vi "UHR-Fleezers Control (host) - 12.8.1.vi"() -> ()   [LabVIEW 2012] (continued)
              }
            }
          }
        }
      }
      event "Stop All": Value Change {
        # "Stopping blue laser before shutting off program"
        n823 = event-data() -> ()  [unwired: 1 in, 5 out]
        n824 = local read "Delay (ms)"() -> (w1275:i32)
        n825 = call "serial write macro.vi"("String"="l0", "Delay (ms)"=w1275, "VISA resource name"=w1278) -> ("read buffer"=w1273:string, "error out"=w1274:errorcluster, "VISA resource name out"=w1277:refnum<visa-resource-name>)
        n826 = local write "read blue buffer"(w1273) -> ()
        n827 = local write "Blue Error Out"(w1274) -> ()
        n828 = VISA Close(VISA resource name=w1277) -> ()  [unwired: 1 in, 1 out]
        n829 = local read "Stop All"() -> (w1279:bool)
      }
    }
    n830 = node-c288() -> ()  [unwired: 1 in, 1 out]
  }
  n831 = node-c288(2 ("Processor")) -> (w78:T27)  [unwired: 3 out]
  n832 = node-c288() -> (w34:T27)  [unwired: 4 out]
  n833 = node-c288() -> (w80:T27)  [unwired: 4 out]
  n834 = while "Duncan's play event loop" {
    stop <- w1281 stop-if-true
    n835 = Create User Event(user event datatype=TRUE ("Boolean")) -> (user event=w1282:refnum<user-event>)  [unwired: 1 in, 1 out]
    n836 = Create User Event(user event datatype=TRUE ("Boolean")) -> (user event=w1289:refnum<user-event>)  [unwired: 1 in, 1 out]
    n837 = global write "Global for fluorescence simulation mean (30 samples), (power series).vi" "Red Signal"(w1282) -> ()
    n838 = global write "Global for fluorescence simulation mean (30 samples), (power series).vi" "Green Signal"(w1289) -> ()
    n839 = register-events(w1289, w1282) -> (reference out=w1288:refnum<event-registration>)  [unwired: 2 in, 1 out]
    n840 = event shown="[1] \"Get Fluorophore\": Value Change" {
      selector: w1288 -> [_ _ _ _]
      dyn-events: _ -> [_ _ _ _]
      timeout: 100 -> [_ _ _ _]
      event Timeout {
        n841 = event-data() -> ()  [unwired: 1 in, 2 out]
      }
      event "Get Fluorophore": Value Change {
        n842 = event-data() -> ("OldVal"=w1291:bool)  [unwired: 1 in, 4 out]
        n843 = case shown="True" w1291 {
          selector: w1291 -> [_ w1292]
          frame False {
          }
          frame True {
            n844 = property on="Move to Position 3" class="Bool"("Val(Sgnl)"=w1292) -> ()  [unwired: 2 in, 2 out]
            n845 = case shown="1" "Numeric" {
              frame 0, Default {
              }
              frame 1 {
                n846 = property on="Green Laser ON" class="Bool (strict)"("Val(Sgnl)"=TRUE ("Value (Signaling)")) -> ()  [unwired: 2 in, 2 out]
              }
              frame 2 {
                n847 = property on="Red Laser ON" class="Bool (strict)"("Val(Sgnl)"=TRUE) -> ()  [unwired: 2 in, 2 out]
              }
            }
          }
        }
      }
      event User Event {
        n848 = event-data() -> ("Boolean"=w1296:bool)  [unwired: 1 in, 3 out]
        "Green Fluorophore" <- w1296
        n849 = property on="Get Fluorophore" class="Bool (strict)"("Val(Sgnl)"=w1296) -> ()  [unwired: 2 in, 2 out]
      }
      event User Event {
        n850 = event-data() -> ("Boolean"=w1297:bool)  [unwired: 1 in, 3 out]
        "Red Fluorophore" <- w1297
        n851 = property on="Get Fluorophore" class="Bool (strict)"("Val(Sgnl)"=w1297) -> ()  [unwired: 2 in, 2 out]
      }
    }
    n852 = property on="Get Fluorophore" class="Bool (strict)"("Val(Sgnl)"="Get Fluorophore") -> ()  [unwired: 2 in, 2 out]
    n853 = Wait (ms)(milliseconds to wait=u32 100) -> ()  [unwired: 1 out]
    n854 = local read "Stop All"() -> (w1280:bool)
    n855 = Or(x=w1280, y="stop") -> (x .or. y?=w1281:bool)
  }
  n856 = timed-loop "Basic control parameters (all FPGA settings, other basic controls)" {
    shift-right: [w1305] -> _
    shift-left: errorcluster {"status"=FALSE, "code"=0, "source"=""} ("error out") -> [_]
    tunnel: [w1304] -> _
    timing: w78 -> [_]
    timing-out: [_] -> w77
    tunnel: w54 -> [w1303]
    tunnel: w44 -> [w1302]
    tunnel: w43 -> [w1301]
    tunnel: w42 -> [w1300]
    tunnel: w41 -> [w1299]
    tunnel: w17 -> [w1298]
    stop <- w1304 stop-if-true
    n857 = node-c288() -> ()  [unwired: 2 out]
    n858 = event shown="[32] \"Read Cal\": Value Change" {
      selector: _ -> [_ _ _ _ _ _ _ _ _ _ _ _ _ _ _ _ _ _ _ _ _ _ _ _ _ _ _ _ _ _ _ _ _ _ _ _ _ _ _ _ _ _ _ _ _ _ _ _ _ _ _ _ _ _ _ _ _ _ _ _ _ _ _ _ _ _ _ _ _ _ _ _ _ _ _]
      dyn-events: _ -> [_ _ _ _ _ _ _ _ _ _ _ _ _ _ _ _ _ _ _ _ _ _ _ _ _ _ _ _ _ _ _ _ _ _ _ _ _ _ _ _ _ _ _ _ _ _ _ _ _ _ _ _ _ _ _ _ _ _ _ _ _ _ _ _ _ _ _ _ _ _ _ _ _ _ _]
      timeout: _ -> [_ _ _ _ _ _ _ _ _ _ _ _ _ _ _ _ _ _ _ _ _ _ _ _ _ _ _ _ _ _ _ _ _ _ _ _ _ _ _ _ _ _ _ _ _ _ _ _ _ _ _ _ _ _ _ _ _ _ _ _ _ _ _ _ _ _ _ _ _ _ _ _ _ _ _]
      tunnel: [w1345 _ _ _ w1375 _ _ _ _ _ _ w1446 _ _ w1514 w1516 w1525 w1527 w1597 _ w1616 w1640 w1660 w1680 w1699 w1723 w1752 _ w1757 w1851 w1855 w1892 _ w1930 w1933 w1936 w1946 w1949 _ w1956 _ _ _ _ _ _ _ _ _ _ _ _ _ _ _ _ _ w2333 _ _ _ _ w2369 _ _ _ _ _ _ _ _ _ _ _ _] -> w1305
      tunnel: [_ _ _ _ _ _ _ _ _ w1431 _ _ _ _ _ _ _ _ _ _ _ _ _ _ _ _ _ _ _ _ _ _ _ _ _ _ _ _ _ _ _ _ _ _ _ _ _ _ _ _ _ _ _ _ _ _ _ _ _ _ _ _ _ _ _ _ _ _ _ _ _ _ _ _ _] -> w1304
      tunnel: [_ _ _ _ _ _ _ "Round T1 X" _ _ _ _ _ _ _ _ _ _ _ _ _ _ _ _ _ _ _ _ _ _ _ _ _ _ _ _ _ _ _ _ _ _ _ _ _ _ _ _ _ _ _ _ _ _ _ _ _ _ _ _ _ _ _ _ _ _ _ _ _ _ _ _ _ _ _] -> _
      tunnel: [_ _ _ "Adjust Scale\nto Mean" _ _ _ _ _ _ _ _ _ _ _ _ _ _ _ _ _ _ _ _ _ _ _ _ "Test ttrig" _ _ _ _ _ _ _ _ _ _ _ _ _ _ _ _ _ _ "Flush Sample" "Flush Pump 3" "Flush Pump 1" "Clear Volume" _ _ _ _ _ _ _ _ _ _ _ _ _ _ _ _ _ _ _ _ _ _ _ _] -> _
      tunnel: [_ _ _ _ _ _ _ _ "Round T2 X" _ "Delayed Interlace Start" _ _ _ _ _ _ _ _ _ _ _ _ _ _ _ _ _ _ _ _ _ _ _ _ _ _ _ _ _ _ _ _ _ _ _ _ _ _ _ _ _ _ _ _ _ _ _ _ _ _ _ _ _ _ _ _ _ _ _ _ _ _ _ _] -> _
      tunnel: w1303 -> [_ _ _ _ _ _ _ _ _ _ _ _ _ _ _ _ _ _ _ _ _ _ _ _ _ _ _ _ _ _ _ _ _ _ _ _ _ _ _ _ _ _ _ w2113 w2120 w2127 w2132 w2141 _ _ w2247 _ _ _ _ _ _ _ _ _ _ _ _ _ _ _ _ _ _ _ _ _ _ _ _]
      tunnel: w1302 -> [_ _ _ _ _ _ _ _ _ _ _ _ _ _ _ _ _ _ _ _ _ _ _ _ _ _ _ _ _ _ _ _ _ _ _ _ _ _ _ _ _ w2030 _ _ _ _ _ _ w2185 _ _ w2253 _ w2262 _ w2276 _ _ _ _ _ _ _ _ _ _ _ _ _ _ _ _ _ _ _]
      tunnel: w1301 -> [_ _ _ _ _ _ _ _ _ _ _ _ _ _ _ _ _ _ _ _ _ _ _ _ _ _ _ _ _ _ _ _ _ _ _ _ _ _ _ _ _ _ _ _ _ _ _ _ _ _ _ _ _ _ _ _ _ _ _ _ _ _ _ _ _ _ _ _ _ _ _ _ _ _ _]
      tunnel: w1300 -> [_ _ _ _ _ _ _ _ _ _ _ _ _ _ _ _ _ _ _ _ _ _ _ _ _ _ _ _ _ _ _ _ _ _ _ _ _ _ _ _ w1967 _ _ _ _ _ _ _ _ w2215 _ _ w2258 _ w2269 _ w2301 _ _ _ _ _ _ _ _ _ _ _ _ _ _ _ _ _ _]
      tunnel: w1299 -> [_ _ _ _ _ _ _ _ _ _ _ _ _ _ _ _ _ _ _ _ _ _ _ _ _ _ _ _ _ _ _ _ _ _ _ _ _ _ _ _ _ _ _ _ _ _ _ _ _ _ _ _ _ _ _ _ _ _ _ _ _ _ _ _ _ _ _ _ _ _ _ _ _ _ _]
      tunnel: w1298 -> [w1308 _ _ _ w1374 _ w1400 _ _ _ _ w1437 _ _ w1492 w1515 w1520 w1526 w1562 _ w1605 w1638 w1641 w1661 w1681 w1700 w1728 w1753 w1755 w1759 w1852 w1856 _ w1927 w1931 w1934 w1944 w1947 _ w1955 _ _ _ _ _ _ _ _ _ _ _ _ _ _ _ _ _ w2326 _ w2347 _ w2353 w2368 _ w2375 w2377 w2384 w2398 w2413 _ w2422 _ w2442 _ _]
      event "AI Count (ticks)", "Sets to FIFO (Traps)", "Save ave N", "FPGA Ave.", "# Samples/channel", "N sets to save": Value Change {
        # "So that if 'Save ave N' is updated, the AOD scanning code updates too."
        n859 = event-data() -> ()  [unwired: 6 out]
        n860 = local read "AI Count (ticks)"() -> (w1329:u16)
        n861 = Unbundle By Name("Sets to FIFO (Traps)") -> ("Set 1"=w1312:bool, "Set 2"=w1311:bool, "Set 3"=w1310:bool)
        n862 = Boolean To (0,1)(Boolean="Sets to FIFO (Traps)") -> (0, 1=w1337:cluster{"Set 1":i16, "Set 2":i16, "Set 3":i16})
        n863 = xnode "Read/Write Control"("FPGA VI Reference In"=w1308, "ai count"=w1329, "Set 1"=w1312, "Set 2"=w1311, "Set 3"=w1310, "N of AI1 Int Acq Sets"="N Acq Sets (Traps + Fl.)") -> ("error out"=w1345:errorcluster)  [unwired: 1 in, 1 out]
        n864 = Cluster To Array(cluster=w1337) -> (array=w1336:i16[])
        n865 = To Unsigned Long Integer(number=w1336) -> (unsigned 32bit integer=w1318:u32[])
        n866 = local read "Scan steps (AOD)"() -> (w1338:u64)
        n867 = Multiply(x=w1329, y="N Acq Sets (Traps + Fl.)") -> (x*y=w1327:u16)
        n868 = Divide(x=40000000.0, y=w1329) -> (x/y=w1321:dbl)
        "AI rate (Hz)" <- w1321
        "Ave. Rate (Hz)" <- w1321
        n869 = Add Array Elements(numeric array=w1318) -> (sum=w1330:u32)
        "Trap Sets" <- w1330
        n870 = Reciprocal(x=w1321) -> (1/x=→"Ave. Period (s)":dbl)
        n871 = property on="Scan steps (AOD)" class="DigNum (strict)"("Val(Sgnl)"=w1338) -> ()  [unwired: 2 in, 2 out]
        n872 = Divide(x=w1321, y="N Acq Sets (Traps + Fl.)") -> (x/y=w1342:dbl)
        "Data Rate (Hz)" <- w1342
        n873 = Reciprocal(x=w1342) -> (1/x=→"Data Period (s)":dbl)
        n874 = local read "Save ave N"() -> (w1341:dbl)
        n875 = Divide(x=w1342, y=w1341) -> (x/y=w1340:dbl)
        "Save Data Rate (Hz)" <- w1340
        n876 = Reciprocal(x=w1340) -> (1/x=→"Save Data Period (s)":dbl)
        n877 = Multiply(x=w1327, y="# Samples/trap") -> (x*y=w1325:u32)
        "Counts/DMA" <- w1325
        n878 = property on="Trap Disp. Downsample" class="DigNum (strict)"("Maximum"="# Samples/trap") -> ()  [unwired: 2 in, 2 out]
        n879 = Multiply(x=w1330, y="# Samples/trap") -> (x*y=w1319:u32)
        "# Samples/channel" <- w1319
        n880 = Multiply(x=w1319, y=u32 8) -> (x*y=→"Trap AI Elements/DMA read":u32)
        n881 = local read "APD Int. Count"() -> (w1326:u32)
        n882 = Multiply(x=w1319, y=u32 3) -> (x*y=→"Trap Pos Elements/DMA read":u32)
        n883 = Divide(x=w1325, y=w1326) -> (x/y=w1316:dbl)
        "APD Samples/FIFO Acq." <- w1316
        n884 = Divide(x=w1325, y=40000000.0) -> (x/y=w1323:dbl)
        "DMA Update Period (s)" <- w1323
        n885 = local read "Number of APDs"() -> (w1309:u8)
        n886 = Multiply(x=w1309, y=w1316) -> (x*y=→"APD Elements/DMA read":dbl)
        n887 = property on="APD Disp. Downsample" class="DigNum (strict)"("Maximum"=w1316) -> ()  [unwired: 2 in, 2 out]
        n888 = local read "N sets to save"() -> (w1335:u32)
        n889 = Multiply(x=w1323, y=w1335) -> (x*y=→"Total Time (s)":dbl)
        "FPGA Averaging" <- FALSE ("FPGA Averaging")
      }
      event "Remove Offset": Value Change {
        n890 = event-data() -> ()  [unwired: 7 out]
        n891 = local write "Remove Offset"(FALSE ("Remove Offset")) -> ()
        n892 = local read "Bead Mean (nm)"() -> (w1347:dbl)
        n893 = local read "Offset (nm)"() -> (w1348:dbl)
        n894 = Add(x=w1347, y=w1348) -> (x+y=w1346:dbl)
        n895 = local write "Offset (nm)"(w1346) -> ()
        n896 = disable-structure shown="Disabled" {
          frame Disabled {
            n897 = local read "Bead Mean (nm)"() -> (w1353:dbl)
            n898 = Add(y=w1353) -> (x=w1352:dbl, x+y=w1351:dbl)
            n899 = Subtract(x=w1353, y=w1352) -> (x-y=w1350:dbl)
            n900 = property on="Bead Separation" class="WFChart (strict)"("YScale.Minimum"=w1350) -> ()  [unwired: 2 in, 2 out]
            n901 = property on="Bead Separation" class="WFChart (strict)"("YScale.Maximum"=w1351) -> ()  [unwired: 2 in, 2 out]
          }
          frame Enabled {
          }
        }
      }
      event "Detector Type": Value Change {
        n902 = event-data() -> ()  [unwired: 7 out]
        n903 = local read "AI labels"() -> (w1355:string[])
        n904 = property on="High Res. Display" class="Ring (strict)"("Strings []"=w1355) -> ()  [unwired: 2 in, 2 out]
        n905 = Build Array (concatenate)(w1355, "none") -> (w1356:string[])
        n906 = property on="FFT 1 Choice 1" class="Ring (strict)"("Strings []"=w1356) -> ()  [unwired: 2 in, 2 out]
        n907 = property on="FFT 1 Choice 2" class="Ring (strict)"("Strings []"=w1356) -> ()  [unwired: 2 in, 2 out]
        n908 = property on="FFT 2 Choice 1" class="Ring (strict)"("Strings []"=w1356) -> ()  [unwired: 2 in, 2 out]
        n909 = property on="FFT 2 Choice 2" class="Ring (strict)"("Strings []"=w1356) -> ()  [unwired: 2 in, 2 out]
        n910 = Bundle("APD 1", "APD 2", "APD 3") -> (w1359:cluster{string, string, string})  [unwired: 1 out]
        n911 = Cluster To Array(cluster=w1359) -> (array=w1357:string[])
        n912 = Build Array (concatenate)(w1357, w1356) -> (w1361:string[])
        n913 = Array Size(array=w1361) -> (size(s)=w1362:i32)
        n914 = property on="Signals to Plot" class="LstBox (strict)"("Item Names"=w1361) -> ()  [unwired: 2 in, 2 out]
        n915 = property on="Signals to Plot" class="LstBox (strict)"("Number of Rows"=w1362) -> ()  [unwired: 2 in, 2 out]
        n916 = property on="All Signals" class="WFChart (strict)"("LegNumRows"=w1362) -> ()  [unwired: 2 in, 2 out]
      }
      event "Adjust Scale\nto Mean": Value Change {
        n917 = event-data() -> ()  [unwired: 7 out]
        n918 = local read "APD 1 Rate (Hz)"() -> (w1371:dbl)
        n919 = Multiply(x=1000.0, y="Above (kHz)") -> (x*y=w1369:dbl)
        n920 = Multiply(x=1000.0, y="Below (kHz)") -> (x*y=w1367:dbl)
        n921 = Add(x=w1369, y=w1371) -> (x+y=w1364:dbl)
        n922 = Subtract(x=w1371, y=w1367) -> (x-y=w1365:dbl)
        n923 = property on="APD Chart" class="WFChart (strict)"("YScale.Minimum"=w1365) -> ()  [unwired: 2 in, 2 out]
        n924 = property on="APD Chart" class="WFChart (strict)"("YScale.Maximum"=w1364) -> ()  [unwired: 2 in, 2 out]
      }
      event "Phase adj. (AI1)", "+ phase (AI1)", "- phase (AI1)": Value Change {
        n925 = event-data() -> ()  [unwired: 7 out]
        n926 = Negate(x="Phase adj. (AI1)") -> (-x=w1382:i16)
        n927 = Select(t=w1382, s="- phase (AI1)", f="Phase adj. (AI1)") -> (s? t:f=w1381:i16)
        n928 = xnode "Read/Write Control"("FPGA VI Reference In"=w1374, "Phase count adjustment"=w1381) -> ("FPGA VI Reference Out"=w1380:T24, "error out"=w1379:errorcluster)  [unwired: 2 in]
        n929 = Or(x="- phase (AI1)", y="+ phase (AI1)") -> (x .or. y?=w1376:bool)
        n930 = xnode "Read/Write Control"("FPGA VI Reference In"=w1380, "error in"=w1379, "+ phase"=w1376) -> ("error out"=w1375:errorcluster)  [unwired: 1 in, 1 out]
      }
      event "Signals to Plot": Double Click {
        w1386 = u32 9868950 ("Color Box")
        n931 = event-data() -> ("Row"=w1388:i32)  [unwired: 9 out]
        n932 = property on="All Signals" class="WFChart (strict)"("Active Plot"=w1388) -> (error out=w1399:errorcluster)  [unwired: 2 in, 1 out]
        n933 = property on="All Signals" class="WFChart (strict)" props=["Plot", "Visible?", "Plot", "Plot Color"](error in=w1399) -> (error out=w1398:errorcluster, "Plot.Visible?"=w1397:bool)  [unwired: 1 in, 2 out]
        n934 = Select(t=FALSE ("Plot.Visible"), s=w1397, f=TRUE ("Plot.Visible")) -> (s? t:f=w1392:bool)
        n935 = property on="All Signals" class="WFChart (strict)"(error in=w1398, "Plot.Visible?"=w1392) -> (error out=w1394:errorcluster)  [unwired: 1 in, 1 out]
        n936 = property on="All Signals" class="WFChart (strict)"(error in=w1394) -> (error out=w1389:errorcluster, "Plot.Plot Color"=w1393:u32)  [unwired: 1 in, 1 out]
        n937 = property on="Signals to Plot" class="LstBox (strict)"(error in=w1389, "Active Row"=w1388) -> (error out=w1387:errorcluster)  [unwired: 1 in, 1 out]
        n938 = Select(t=w1393, s=w1392, f=u32 0) -> (s? t:f=w1390:u32)
        n939 = property on="Signals to Plot" class="LstBox (strict)"(error in=w1387, "CellFontColor"=w1390, "SelColor"=w1386, "CellBG"=w1386, "CellFontSize"=u32 20 ("Active Row:Cell Font:Size"), "CellFontBold"=TRUE ("Active Row:Cell Font:Bold")) -> ()  [unwired: 1 in, 2 out]
      }
      event "BD 1 Frequency 1 (MHz)", "BD 1 Frequency 2 (MHz)", "BD 1 Frequency 3 (MHz)", "BD 2 Frequency 1 (MHz)", "BD 2 Frequency 2 (MHz)", "BD 2 Frequency 3 (MHz)", "Trap Delta (MHz)", "Update all trap values": Value Change {
        # "This is so you can set trap frequencies\nvia local variables and then update\nall at once"
        n940 = event-data() -> ("CtlRef"=w1404:refnum<vi>)  [unwired: 6 out]
        n941 = control-ref of="Trap Delta (MHz)"() -> (w1403:refnum<vi>)
        n942 = Equal?(x=w1403, y=w1404) -> (x = y?=w1402:bool)
        n943 = local write "Update all trap values"(FALSE ("Update all trap values")) -> ()
        n944 = case shown="False" "Oscillate Set 1" {
          tunnel: w1402 -> [w1408 _]
          tunnel: w1400 -> [w1406 _]
          frame False {
            n945 = local read "BD 1 Frequency 2 (MHz)"() -> (w1412:dbl)
            n946 = local read "BD 1 Frequency 1 (MHz)"() -> (w1410:dbl)
            n947 = Subtract(x=w1412, y="Trap Delta (MHz)") -> (x-y=w1409:dbl)
            n948 = Select(t=w1409, s=w1408, f=w1410) -> (s? t:f=w1407:dbl)
            n949 = local read "Y RF Frequency Limits (MHz)"() -> (w1413:T18)
            n950 = local read "X RF Frequency Limits (MHz)"() -> (w1414:T18)
            n951 = local write "BD 1 Frequency 1 (MHz)"(w1407) -> ()
            n952 = local read "BD 1 Frequency 3 (MHz)"() -> (w1423:dbl)
            n953 = local read "BD 2 Frequency 1 (MHz)"() -> (w1417:dbl)
            n954 = local read "BD 2 Frequency 2 (MHz)"() -> (w1416:dbl)
            n955 = local read "BD 2 Frequency 3 (MHz)"() -> (w1424:dbl)
            n956 = call "set RF board frequency - interlace.vi"("Board 2 Frequency Limits"=w1413, "Board 1 Frequency Limits"=w1414, "FPGA VI Reference In"=w1406, "Board 2 Frequency 3 (MHz)"=w1424, "Board 1 Frequency 3 (MHz)"=w1423, "Board 2 Frequency 2 (MHz)"=w1416, "Board 2 Frequency 1 (MHz)"=w1417, "Board 1 Frequency 2 (MHz)"=w1412, "Board 1 Frequency 1  (MHz)"=w1407) -> ()  [unwired: 1 in, 2 out]
            n957 = Subtract(x=w1417, y=w1416) -> (x-y=w1421:dbl)
            n958 = Subtract(x=w1407, y=w1412) -> (x-y=w1422:dbl)
            n959 = Square(x=w1421) -> (x^2=w1419:dbl)
            n960 = Square(x=w1422) -> (x^2=w1420:dbl)
            n961 = Add(x=w1420, y=w1419) -> (x+y=w1418:dbl)
            n962 = Square Root(x=w1418) -> (sqrt(x)=w1415:dbl)
            n963 = property on="Initial delta (MHz)" class="DigNum (strict)"("Val(Sgnl)"=w1415) -> ()  [unwired: 2 in, 2 out]
            n964 = local write "Trap Delta (MHz)"(w1415) -> ()
          }
          frame True {
          }
        }
      }
      event "Round T1 X": Value Change {
        n965 = event-data() -> ()  [unwired: 7 out]
        n966 = local read "BD 1 Frequency 1 (MHz)"() -> (w1427:dbl)
        n967 = Round To Nearest(number=w1427) -> (nearest integer value=w1426:dbl)
        n968 = property on="BD 1 Frequency 1 (MHz)" class="DigNum (strict)"("Val(Sgnl)"=w1426) -> ()  [unwired: 2 in, 2 out]
      }
      event "Round T2 X": Value Change {
        n969 = event-data() -> ()  [unwired: 7 out]
        n970 = local read "BD 1 Frequency 2 (MHz)"() -> (w1429:dbl)
        n971 = Round To Nearest(number=w1429) -> (nearest integer value=w1428:dbl)
        n972 = property on="BD 1 Frequency 2 (MHz)" class="DigNum (strict)"("Val(Sgnl)"=w1428) -> ()  [unwired: 2 in, 2 out]
      }
      event "Stop All": Value Change {
        n973 = event-data() -> ()  [unwired: 7 out]
        n974 = local read "Stop All"() -> (w1431:bool)
      }
      event "Delayed Interlace Start": Value Change {
        n975 = event-data() -> ()  [unwired: 7 out]
        n976 = flat-sequence {
          frame #0 {
            n977 = Multiply(x="Delay to Interlace (s)", y=1000.0) -> (x*y=w1433:dbl)
            n978 = Wait (ms)(milliseconds to wait=w1433) -> ()  [unwired: 1 out]
          }
          frame #1 {
            n979 = property on="Laser interlacing mode" class="RadioBtnsControl (strict)"("Val(Sgnl)"=enum32{"Laser ON", "Laser OFF", "Interlace"}."Interlace" ("Value (Signaling)")) -> ()  [unwired: 2 in, 2 out]
          }
        }
      }
      event "BD 1 Amplitude 1 (%)", "BD 1 Amplitude 2 (%)", "BD 1 Amplitude 3 (%)", "BD 2 Amplitude 1 (%)", "BD 2 Amplitude 2 (%)", "BD 2 Amplitude 3 (%)", "Trap 1 ON", "Trap 2 ON", "Trap 3 ON", "Feedback On/Off", "All FB On/Off": Value Change {
        w1458 = i16 1 ("f")
        n980 = event-data() -> ()  [unwired: 7 out]
        n981 = local write "Trap 1 (ON/OFF)"("Trap 1 ON") -> ()
        n982 = local write "Trap 2 (ON/OFF)"("Trap 2 ON") -> ()
        n983 = Boolean To (0,1)(Boolean="Trap 3 ON") -> (0, 1=w1459:i16)
        n984 = Boolean To (0,1)(Boolean="Trap 1 ON") -> (0, 1=w1460:i16)
        n985 = Boolean To (0,1)(Boolean="Trap 2 ON") -> (0, 1=w1461:i16)
        n986 = Select(t=w1461, s="Trap ON/OFF X or Y Amp?", f=w1458) -> (s? t:f=w1456:i16)
        n987 = Select(t=w1460, s="Trap ON/OFF X or Y Amp?", f=w1458) -> (s? t:f=w1457:i16)
        n988 = Select(t=w1459, s="Trap ON/OFF X or Y Amp?", f=w1458) -> (s? t:f=w1455:i16)
        n989 = Select(t=w1458, s="Trap ON/OFF X or Y Amp?", f=w1461) -> (s? t:f=w1453:i16)
        n990 = Select(t=w1458, s="Trap ON/OFF X or Y Amp?", f=w1460) -> (s? t:f=w1454:i16)
        n991 = Select(t=w1458, s="Trap ON/OFF X or Y Amp?", f=w1459) -> (s? t:f=w1452:i16)
        n992 = And(x="All FB On/Off", y="Feedback On/Off") -> (x .and. y?=w1450:cluster{"Set 1":bool, "Set 2":bool})
        n993 = local read "BD 1 Amplitude 1 (%)"() -> (w1468:dbl)
        n994 = local read "BD 1 Amplitude 2 (%)"() -> (w1467:dbl)
        n995 = local read "BD 1 Amplitude 3 (%)"() -> (w1466:dbl)
        n996 = Unbundle By Name(w1450) -> ("Set 1"=w1445:bool, "Set 2"=w1442:bool)
        n997 = local read "Y RF Amplitude Limits (%)"() -> (w1438:T18)
        n998 = local read "X RF Amplitude Limits (%)"() -> (w1439:T18)
        n999 = local read "BD 2 Amplitude 1 (%)"() -> (w1469:dbl)
        n1000 = local read "BD 2 Amplitude 2 (%)"() -> (w1470:dbl)
        n1001 = local read "BD 2 Amplitude 3 (%)"() -> (w1471:dbl)
        n1002 = And(x="Trap 2 ON", y=w1442) -> (x .and. y?=w1440:bool)
        n1003 = And(x="Trap 1 ON", y=w1445) -> (x .and. y?=w1443:bool)
        n1004 = Multiply(x=w1457, y=w1468) -> (x*y=w1465:dbl)
        n1005 = Multiply(x=w1467, y=w1456) -> (x*y=w1463:dbl)
        n1006 = Multiply(x=w1466, y=w1455) -> (x*y=w1464:dbl)
        n1007 = Multiply(x=w1469, y=w1454) -> (x*y=w1472:dbl)
        n1008 = Multiply(x=w1470, y=w1453) -> (x*y=w1473:dbl)
        n1009 = Multiply(x=w1471, y=w1452) -> (x*y=w1474:dbl)
        n1010 = call "set RF board amplitude - interlace.vi"("Board 2 Amplitude Limits"=w1438, "Board 1 Amplitude Limits"=w1439, "FPGA VI Reference In"=w1437, "Board 2 Amplitude 3 (%)"=w1474, "Board 1 Amplitude 3 (%)"=w1464, "Board 2 Amplitude 2 (%)"=w1473, "Board 2 Amplitude 1 (%)"=w1472, "Board 1 Amplitude 2 (%)"=w1463, "Board 1 Amplitude 1 (%)"=w1465) -> ("error out"=w1447:errorcluster, "FPGA VI Reference Out"=w1448:T24)  [unwired: 1 in]
        n1011 = xnode "Read/Write Control"("FPGA VI Reference In"=w1448, "error in"=w1447, "FB On/Off Set 1"=w1443, "FB On/Off Set 2"=w1440) -> ("error out"=w1446:errorcluster)  [unwired: 1 out]
      }
      event "Load parameters": Value Change {
        n1012 = event-data() -> ()  [unwired: 7 out]
        n1013 = property on="Saved AOD Raster Scan Parameter Sets" class="Arr (strict)"() -> ("Index Values"=w1485:u32[])  [unwired: 2 in, 2 out]
        n1014 = Index Array(array=w1485, index=0) -> (element=w1482:u32)
        n1015 = local write "Load parameters"(FALSE ("Load parameters")) -> ()
        n1016 = Index Array(array="Saved AOD Raster Scan Parameter Sets", index=w1482) -> (element=w1481:T34)
        n1017 = Unbundle By Name(w1481) -> ("Scan Range AOD (nm) 2"=w1480:dbl, "Step Size AOD (nm) 2"=w1479:dbl, "Scan Speed AOD (nm/s) 2"=w1478:dbl, "Number of scans (AOD) 2"=w1477:u16)
        n1018 = flat-sequence {
          tunnel: w1480 -> [w1488]
          tunnel: w1479 -> [w1487]
          tunnel: w1478 -> [w1486]
          tunnel: w1477 -> [w1489]
          frame #0 {
            n1019 = local write "Scan Speed (nm/s)"(w1486) -> ()
            n1020 = local write "Scan Range (nm)"(w1488) -> ()
            n1021 = local write "Step Size (nm)"(w1487) -> ()
          }
          frame #1 {
            n1022 = property on="Number of F/B Scans (AOD)" class="DigNum (strict)"("Val(Sgnl)"=w1489) -> ()  [unwired: 2 in, 2 out]
          }
        }
      }
      event "Trap 1 (ON/OFF)", "Trap 2 (ON/OFF)": Value Change {
        n1023 = event-data() -> ()  [unwired: 7 out]
        n1024 = property on="Trap 2 ON" class="Bool (strict)"("Val(Sgnl)"="Trap 2 (ON/OFF)") -> ()  [unwired: 2 in, 2 out]
        n1025 = property on="Trap 1 ON" class="Bool (strict)"("Val(Sgnl)"="Trap 1 (ON/OFF)") -> ()  [unwired: 2 in, 2 out]
      }
      event "DIO count 1 (ticks)", "DIO count 2 (ticks)", "DIO count 3 (ticks)", "Interlace", "Number Interlace Sets", "Not-Interlacing Set", "BD 1 Delay (ticks)", "BD 2 Delay (Ticks)", "Next trap write delay (ticks)", "XY phase ext loop method", "Amp switch delay 2", "BD 2 Delay (Ticks) 2", "BD 1 Delay (ticks) 2": Value Change {
        n1026 = event-data() -> ()  [unwired: 7 out]
        n1027 = local read "DIO count 3 (ticks)"() -> (w1510:u16)
        n1028 = local read "DIO count 1 (ticks)"() -> (w1512:u16)
        n1029 = local read "DIO count 2 (ticks)"() -> (w1511:u16)
        n1030 = To Unsigned Byte Integer(number="Not-Interlacing Set") -> (unsigned 8bit integer=w1501:u8)
        n1031 = Add(x=w1501, y=u8 1) -> (x+y=w1505:u8)
        n1032 = xnode "Read/Write Control"("FPGA VI Reference In"=w1492, "DIO count 1 (ticks)"=w1512, "DIO count 2 (ticks)"=w1511, "DIO count 3 (ticks)"=w1510, "Interlace ON/OFF"="Interlace", "Number Interlace Cycles"="Number Interlace Sets", "Interlace Off Parameters"=w1505, "BD 1 Delay (ticks)"="BD 1 Delay (ticks)", "BD 2 Delay (Ticks)"="BD 2 Delay (Ticks)", "Next trap write delay (ticks)"="Next trap write delay (ticks)", "XY phase ext loop method"="XY phase ext loop method", "Amp switch delay 2"="Amp switch delay 2", "BD 2 Delay (Ticks) 2"="BD 2 Delay (Ticks) 2", "BD 1 Delay (ticks) 2"="BD 1 Delay (ticks) 2") -> ("error out"=w1514:errorcluster)  [unwired: 1 in, 1 out]
        n1033 = Build Array(w1512, w1511, w1510) -> (w1503:u16[])
        n1034 = Split 1D Array(array=w1503, index="Number Interlace Sets") -> (first subarray=w1513:u16[])  [unwired: 1 out]
        n1035 = Index Array(array=w1503, index=w1501) -> (element=w1502:u16)
        n1036 = Add Array Elements(numeric array=w1513) -> (sum=w1507:u16)
        n1037 = Select(t=w1507, s="Interlace", f=w1502) -> (s? t:f=→"Total Counts (ticks)":u16)
      }
      event "Reset Feedback": Value Change {
        n1038 = event-data() -> ()  [unwired: 7 out]
        n1039 = Unbundle By Name("Reset Feedback") -> ("Set 1"=w1518:bool, "Set 2"=w1517:bool)
        n1040 = xnode "Read/Write Control"("FPGA VI Reference In"=w1515, "FB Reset Set 1"=w1518, "FB Reset Set 2"=w1517) -> ("error out"=w1516:errorcluster)  [unwired: 1 in, 1 out]
      }
      event "Trap Intensity PID Gains": Value Change {
        n1041 = event-data() -> ()  [unwired: 7 out]
        n1042 = Unbundle By Name("Trap Intensity PID Gains") -> ("proportional gain (Kc)"=w1523:i16, "integral gain (Kc*Ts/Ti)"=w1522:i16, "derivative gain (Kc*Td/Ts)"=w1521:i16)
        n1043 = xnode "Read/Write Control"("FPGA VI Reference In"=w1520, "P1"=w1523, "I1"=w1522, "D1"=w1521) -> ("error out"=w1525:errorcluster)  [unwired: 1 in, 1 out]
      }
      event "AI2 to Setpoint", "Setpoints (V)": Value Change {
        n1044 = event-data() -> ()  [unwired: 7 out]
        n1045 = xnode "Read/Write Control"("FPGA VI Reference In"=w1526) -> ("FPGA VI Reference Out"=w1529:T24, "error out"=w1528:errorcluster, "AI2 Y Sum Set 1"=w1536:i16, "AI2 Y Sum Set 2"=w1535:i16)  [unwired: 1 in]
        n1046 = Cluster To Array(cluster="AI2 to Setpoint") -> (array=w1539:bool[])
        n1047 = local read "AI2 (V)"() -> (w1537:cluster{"Set 1":dbl, "Set 2":dbl})
        n1048 = Or Array Elements(Boolean array=w1539) -> (logical OR=w1540:bool)
        n1049 = Bundle By Name(cluster=w1537, "Set 1"=w1536, "Set 2"=w1535) -> (w1534:cluster{"Set 1":dbl, "Set 2":dbl})
        n1050 = Divide(x=w1534, y=3276.7) -> (x/y=w1533:cluster{"Set 1":dbl, "Set 2":dbl})
        "AI2 (V)" <- w1533
        n1051 = case shown="True" w1540 {
          tunnel: [w1543 w1560] -> w1532
          tunnel: "AI2 to Setpoint" -> [_ w1556]
          tunnel: "Setpoints (V)" -> [w1544 w1559]
          tunnel: w1533 -> [_ w1553]
          frame False {
            n1052 = Multiply(x=3276.7, y=w1544) -> (x*y=w1545:cluster{"Set 1":dbl, "Set 2":dbl})
            n1053 = To Word Integer(number=w1545) -> (16bit integer=w1543:cluster{"Set 1":i16, "Set 2":i16})
          }
          frame True {
            n1054 = Unbundle By Name(w1553) -> ("Set 1"=w1552:dbl, "Set 2"=w1551:dbl)
            n1055 = Unbundle By Name(w1559) -> ("Set 1"=w1558:dbl, "Set 2"=w1557:dbl)
            n1056 = Unbundle By Name(w1556) -> ("Set 1"=w1555:bool, "Set 2"=w1554:bool)
            n1057 = Select(t=w1552, s=w1555, f=w1558) -> (s? t:f=w1550:dbl)
            n1058 = Select(t=w1551, s=w1554, f=w1557) -> (s? t:f=w1549:dbl)
            n1059 = Bundle By Name(cluster=w1559, "Set 1"=w1550, "Set 2"=w1549) -> (w1547:cluster{"Set 1":dbl, "Set 2":dbl})
            n1060 = local write "Setpoints (V)"(w1547) -> ()
            n1061 = Multiply(x=3276.7, y=w1547) -> (x*y=w1548:cluster{"Set 1":dbl, "Set 2":dbl})
            n1062 = To Word Integer(number=w1548) -> (16bit integer=w1560:cluster{"Set 1":i16, "Set 2":i16})
          }
        }
        n1063 = Unbundle By Name(w1532) -> ("Set 1"=w1531:i16, "Set 2"=w1530:i16)
        n1064 = xnode "Read/Write Control"("FPGA VI Reference In"=w1529, "error in"=w1528, "FB Setpoint Set 1"=w1531, "FB Setpoint Set 2"=w1530) -> ("error out"=w1527:errorcluster)  [unwired: 1 out]
      }
      event "+ phase (GI)", "- phase (GI)", "+ phase (GI) 2", "- phase (GI) 2", "+ phase (RI)", "- phase (RI)", "+ phase (Green FB)", "- phase (Green FB)": Value Change {
        n1065 = event-data() -> ()  [unwired: 7 out]
        n1066 = Or(x="+ phase (GI)", y="- phase (GI)") -> (x .or. y?=w1596:bool)
        n1067 = Negate(x="Phase adj. (GI)") -> (-x=w1601:i16)
        n1068 = Select(t=w1601, s="+ phase (GI)", f="Phase adj. (GI)") -> (s? t:f=w1600:i16)
        n1069 = Or(x="+ phase (GI) 2", y="- phase (GI) 2") -> (x .or. y?=w1587:bool)
        n1070 = Negate(x="Phase adj. (GI) 2") -> (-x=w1592:i16)
        n1071 = Select(t=w1592, s="+ phase (GI) 2", f="Phase adj. (GI) 2") -> (s? t:f=w1588:i16)
        n1072 = Negate(x="Phase adj. (RI)") -> (-x=w1586:i16)
        n1073 = Or(x="+ phase (RI)", y="- phase (RI)") -> (x .or. y?=w1582:bool)
        n1074 = Select(t=w1586, s="+ phase (RI)", f="Phase adj. (RI)") -> (s? t:f=w1581:i16)
        n1075 = Or(x="+ phase (Green FB)", y="- phase (Green FB)") -> (x .or. y?=w1575:bool)
        n1076 = Negate(x="Phase adj. (Green FB)") -> (-x=w1580:i16)
        n1077 = Select(t=w1580, s="+ phase (Green FB)", f="Phase adj. (Green FB)") -> (s? t:f=w1576:i16)
        n1078 = Negate(x="Phase adj. (BI AO)") -> (-x=w1574:i16)
        n1079 = Or(x="+ phase (BI AO)", y="- phase (BI AO)") -> (x .or. y?=w1564:bool)
        n1080 = Select(t=w1574, s="+ phase (BI AO)", f="Phase adj. (BI AO)") -> (s? t:f=w1566:i16)
        n1081 = Negate(x="Phase adj. (BI DO)") -> (-x=w1570:i16)
        n1082 = Or(x="+ phase (BI DO)", y="- phase (BI DO)") -> (x .or. y?=w1563:bool)
        n1083 = Select(t=w1570, s="+ phase (BI DO)", f="Phase adj. (BI DO)") -> (s? t:f=w1565:i16)
        n1084 = xnode "Read/Write Control"("FPGA VI Reference In"=w1562, "Phase count adjustment (GI)"=w1600, "Phase count adjustment (GI) 2"=w1588, "Phase count adjustment (RI)"=w1581, "Phase count adjustment (Green FB)"=w1576, "Phase count adjustment (BI AO)"=w1566, "Phase count adjustment (BI D)"=w1565) -> ("FPGA VI Reference Out"=w1598:T24, "error out"=w1599:errorcluster)  [unwired: 1 in]
        n1085 = xnode "Read/Write Control"("FPGA VI Reference In"=w1598, "error in"=w1599, "+ phase (GI)"=w1596, "+ phase (GI) 2"=w1587, "+ phase (RI)"=w1582, "+ phase (Green FB)"=w1575, "+ phase (BI AO)"=w1564, "+ phase (BI D)"=w1563) -> ("error out"=w1597:errorcluster)  [unwired: 1 out]
      }
      event "Green Laser ON/OFF", "Red Laser ON/OFF", "Blue Laser ON/OFF": Value Change {
        # "This loop shouldn't be initialized.  The main 'laser ON' settings should dominate and set the others."
        n1086 = event-data() -> ()  [unwired: 7 out]
        n1087 = property on="Red Laser ON" class="Bool (strict)"("Val(Sgnl)"="Red Laser ON/OFF") -> ()  [unwired: 2 in, 2 out]
        n1088 = property on="Blue Laser ON" class="Bool (strict)"("Val(Sgnl)"="Blue Laser ON/OFF") -> ()  [unwired: 2 in, 2 out]
        n1089 = property on="Green Laser ON" class="Bool (strict)"("Val(Sgnl)"="Green Laser ON/OFF") -> ()  [unwired: 2 in, 2 out]
      }
      event "Laser interlacing mode", "Green Laser ON", "Red Laser ON", "Blue Laser ON": Value Change {
        n1090 = event-data() -> ()  [unwired: 7 out]
        n1091 = local write "Green Laser ON/OFF"("Green Laser ON") -> ()
        n1092 = local write "Blue Laser ON/OFF"("Blue Laser ON") -> ()
        n1093 = local write "Red Laser ON/OFF"("Red Laser ON") -> ()
        n1094 = case shown="True" "Green Laser ON" {
          tunnel: "Laser interlacing mode" -> [_ w1637]
          tunnel: [enum32{"Laser ON", "Laser OFF", "Interlace"}."Laser OFF" ("Green laser mode") w1637] -> w1615
          tunnel: [FALSE w1633] -> w1614
          frame False {
          }
          frame True {
            n1095 = local read "Green FB On/Off"() -> (w1634:bool)
            n1096 = Equal?(x=w1637, y=enum32{"Laser ON", "Laser OFF", "Interlace"}."Interlace") -> (x = y?=w1635:bool)
            n1097 = And(x=w1635, y=w1634) -> (x .and. y?=w1633:bool)
          }
        }
        n1098 = case shown="True" "Red Laser ON" {
          tunnel: "Laser interlacing mode" -> [_ w1630]
          tunnel: [enum32{"Laser ON", "Laser OFF", "Interlace"}."Laser OFF" ("Green laser mode") w1630] -> w1611
          tunnel: [FALSE w1626] -> w1610
          frame False {
          }
          frame True {
            n1099 = local read "Red FB On/Off"() -> (w1627:bool)
            n1100 = Equal?(x=w1630, y=enum32{"Laser ON", "Laser OFF", "Interlace"}."Interlace") -> (x = y?=w1628:bool)
            n1101 = And(x=w1628, y=w1627) -> (x .and. y?=w1626:bool)
          }
        }
        n1102 = case shown="True" "Blue Laser ON" {
          tunnel: "Laser interlacing mode" -> [_ w1621]
          tunnel: [enum32{"Laser ON", "Laser OFF", "Interlace"}."Laser OFF" ("Green laser mode") w1621] -> w1607
          tunnel: [FALSE w1619] -> w1606
          frame False {
          }
          frame True {
            n1103 = local read "Blue FB On/Off"() -> (w1620:bool)
            n1104 = Equal?(x=w1621, y=enum32{"Laser ON", "Laser OFF", "Interlace"}."Interlace") -> (x = y?=w1622:bool)
            n1105 = And(x=w1622, y=w1620) -> (x .and. y?=w1619:bool)
          }
        }
        n1106 = xnode "Read/Write Control"("FPGA VI Reference In"=w1605, "Operating Mode"=w1615, "Operating Mode 2"=w1615, "Green FB On/Off"=w1614, "Red Laser Operating Mode"=w1611, "RI Operating Mode 2"=w1611, "Red FB On/Off"=w1610, "BI Operating Mode (AO)"=w1607, "Blue Laser Operating Mode (D)"=w1607, "Blue FB On/Off"=w1606) -> ("error out"=w1616:errorcluster)  [unwired: 1 in, 1 out]
      }
      event "Invert laser interlacing": Value Change {
        n1107 = event-data() -> ()  [unwired: 7 out]
        n1108 = xnode "Read/Write Control"("FPGA VI Reference In"=w1638, "Invert GI"="Invert laser interlacing", "Invert GI 2"="Invert laser interlacing", "Invert RI"="Invert laser interlacing", "Invert RI 2"="Invert laser interlacing", "Invert BI (AO)"="Invert laser interlacing", "Invert BI (D)"="Invert laser interlacing") -> ("error out"=w1640:errorcluster)  [unwired: 1 in, 1 out]
      }
      event "Green FB Setpoint (mV)", "Green FB Gains", "Green FB On/Off", "Green Intensity % (FB OFF)", "Green int current ON count adj": Value Change {
        n1109 = event-data() -> ()  [unwired: 7 out]
        n1110 = local read "Green FB Setpoint (mV)"() -> (w1652:dbl)
        n1111 = Multiply(x=w1652, y=3.2767) -> (x*y=w1651:dbl)
        n1112 = local read "Green Intensity % (FB OFF)"() -> (w1655:dbl)
        n1113 = Multiply(x=w1655, y=655.35) -> (x*y=w1656:dbl)
        n1114 = To Unsigned Word Integer(number=w1656) -> (unsigned 16bit integer=w1654:u16)
        n1115 = local read "Green int current ON count adj"() -> (w1658:u32)
        n1116 = local read "Laser interlacing mode"() -> (w1648:enum32{"Laser ON", "Laser OFF", "Interlace"})
        n1117 = local read "Green FB Gains"() -> (w1645:T11)
        n1118 = local read "Green Laser ON"() -> (w1649:bool)
        n1119 = local read "Green FB On/Off"() -> (w1659:bool)
        n1120 = Equal?(x=w1648, y=enum32{"Laser ON", "Laser OFF", "Interlace"}."Interlace") -> (x = y?=w1646:bool)
        n1121 = Unbundle By Name(w1645) -> ("proportional gain (Kc)"=w1644:i16, "integral gain (Kc*Ts/Ti)"=w1643:i16, "derivative gain (Kc*Td/Ts)"=w1642:i16)
        n1122 = Compound Arithmetic op=AND(w1646, w1659, w1649) -> (w1650:bool)
        n1123 = xnode "Read/Write Control"("FPGA VI Reference In"=w1641, "Green FB Setpoint"=w1651, "Green FB On/Off"=w1650, "Current Out"=w1654, "Green int current ON count adj"=w1658, "P3"=w1644, "I3"=w1643, "D3"=w1642) -> ("error out"=w1660:errorcluster)  [unwired: 1 in, 1 out]
      }
      event "Blue FB Setpoint (mV)", "Blue FB Gains", "Blue FB On/Off", "Blue Intensity % (FB OFF)", "Blue int AO ON count adjust": Value Change {
        # "16 bit analog out"
        n1124 = event-data() -> ()  [unwired: 7 out]
        n1125 = Multiply(x="Blue FB Setpoint (mV)", y=3.2767) -> (x*y=w1675:dbl)
        n1126 = Multiply(x="Blue Intensity % (FB OFF)", y=655.35) -> (x*y=w1678:dbl)
        n1127 = To Unsigned Word Integer(number=w1678) -> (unsigned 16bit integer=w1677:u16)
        n1128 = local read "Laser interlacing mode"() -> (w1673:enum32{"Laser ON", "Laser OFF", "Interlace"})
        n1129 = Unbundle By Name("Blue FB Gains") -> ("proportional gain (Kc)"=w1670:i16, "integral gain (Kc*Ts/Ti)"=w1669:i16, "derivative gain (Kc*Td/Ts)"=w1668:i16)
        n1130 = local read "Blue Laser ON"() -> (w1662:bool)
        n1131 = Equal?(x=w1673, y=enum32{"Laser ON", "Laser OFF", "Interlace"}."Interlace") -> (x = y?=w1671:bool)
        n1132 = Compound Arithmetic op=AND(w1671, "Blue FB On/Off", w1662) -> (w1674:bool)
        n1133 = xnode "Read/Write Control"("FPGA VI Reference In"=w1661, "Blue FB Setpoint"=w1675, "Blue FB On/Off"=w1674, "BI Current Out"=w1677, "Blue current ON count adj (AO)"="Blue int AO ON count adjust", "P5"=w1670, "I5"=w1669, "D5"=w1668) -> ("error out"=w1680:errorcluster)  [unwired: 1 in, 1 out]
      }
      event "Red FB Setpoint (mV)", "Red FB Gains", "Red FB On/Off", "Red Intensity % (FB OFF)": Value Change {
        n1134 = event-data() -> ()  [unwired: 7 out]
        n1135 = local read "Red FB Setpoint (mV)"() -> (w1693:dbl)
        n1136 = Multiply(x=w1693, y=3.2767) -> (x*y=w1692:dbl)
        n1137 = local read "Red Intensity % (FB OFF)"() -> (w1682:dbl)
        n1138 = Multiply(x=w1682, y=655.35) -> (x*y=w1696:dbl)
        n1139 = To Unsigned Word Integer(number=w1696) -> (unsigned 16bit integer=w1695:u16)
        n1140 = local read "Laser interlacing mode"() -> (w1689:enum32{"Laser ON", "Laser OFF", "Interlace"})
        n1141 = local read "Red FB Gains"() -> (w1686:T11)
        n1142 = local read "Red Laser ON"() -> (w1690:bool)
        n1143 = local read "Red FB On/Off"() -> (w1698:bool)
        n1144 = Equal?(x=w1689, y=enum32{"Laser ON", "Laser OFF", "Interlace"}."Interlace") -> (x = y?=w1687:bool)
        n1145 = Unbundle By Name(w1686) -> ("proportional gain (Kc)"=w1685:i16, "integral gain (Kc*Ts/Ti)"=w1684:i16, "derivative gain (Kc*Td/Ts)"=w1683:i16)
        n1146 = Compound Arithmetic op=AND(w1687, w1698, w1690) -> (w1691:bool)
        n1147 = xnode "Read/Write Control"("FPGA VI Reference In"=w1681, "Red FB Setpoint"=w1692, "Red FB On/Off"=w1691, "RI Current Out"=w1695, "P4"=w1685, "I4"=w1684, "D4"=w1683) -> ("error out"=w1699:errorcluster)  [unwired: 1 in, 1 out]
      }
      event "+ phase (APD 1 Gate)", "- phase (APD 1 Gate)", "+ phase (APD 2 Gate)", "- phase (APD 2 Gate)", "+ phase (APD 3 Gate)", "- phase (APD 3 Gate)", "+ phase (APD Acq)", "- phase (APD Acq)": Value Change {
        n1148 = event-data() -> ()  [unwired: 7 out]
        n1149 = local read "Phase Adj. (APD 1 Gate)"() -> (w1720:i16)
        n1150 = Or(x="- phase (APD 1 Gate)", y="+ phase (APD 1 Gate)") -> (x .or. y?=w1722:bool)
        n1151 = Negate(x=w1720) -> (-x=w1727:i16)
        n1152 = Select(t=w1727, s="+ phase (APD 1 Gate)", f=w1720) -> (s? t:f=w1726:i16)
        n1153 = local read "Phase Adj. (APD 2 Gate)"() -> (w1717:i16)
        n1154 = Or(x="- phase (APD 2 Gate)", y="+ phase (APD 2 Gate)") -> (x .or. y?=w1715:bool)
        n1155 = Negate(x=w1717) -> (-x=w1719:i16)
        n1156 = Select(t=w1719, s="+ phase (APD 2 Gate)", f=w1717) -> (s? t:f=w1716:i16)
        n1157 = Negate(x="Phase Adj. (APD 3 Gate)") -> (-x=w1714:i16)
        n1158 = Or(x="- phase (APD 3 Gate)", y="+ phase (APD 3 Gate)") -> (x .or. y?=w1710:bool)
        n1159 = Select(t=w1714, s="+ phase (APD 3 Gate)", f="Phase Adj. (APD 3 Gate)") -> (s? t:f=w1711:i16)
        n1160 = local read "Phase Adj. (APD Acq)"() -> (w1708:i16)
        n1161 = Or(x="- phase (APD Acq)", y="+ phase (APD Acq)") -> (x .or. y?=w1706:bool)
        n1162 = Negate(x=w1708) -> (-x=w1709:i16)
        n1163 = Select(t=w1709, s="+ phase (APD Acq)", f=w1708) -> (s? t:f=w1707:i16)
        n1164 = xnode "Read/Write Control"("FPGA VI Reference In"=w1700, "Phase count adjustment (APD 1 Gate)"=w1726, "Phase count adjustment (APD 2 Gate)"=w1716, "Phase count adjustment (APD 3 Gate)"=w1711, "Phase Count Adjustment (APD Acq)"=w1707) -> ("FPGA VI Reference Out"=w1724:T24, "error out"=w1725:errorcluster)  [unwired: 1 in]
        n1165 = xnode "Read/Write Control"("FPGA VI Reference In"=w1724, "error in"=w1725, "+ phase (APD 1 Gate)"=w1722, "+ phase (APD 2 Gate)"=w1715, "+ phase (APD 3 Gate)"=w1710, "+ phase (APD Acq)"=w1706) -> ("error out"=w1723:errorcluster)  [unwired: 1 out]
      }
      event "Invert APD Gate", "APD Gate ON Count", "APD Gate OFF Count", "APD Gate", "APD Integration Time (s)", "APD AO Scale Factor", "Duty Frequency (ON 1/N cycles)", "Interlace ON count", "Interlace OFF count": Value Change {
        n1166 = event-data() -> ()  [unwired: 7 out]
        n1167 = Add(x="Interlace ON count", y="Interlace OFF count") -> (x+y=w1734:u16)
        n1168 = Add(x="APD Gate ON Count", y="APD Gate OFF Count") -> (x+y=w1745:u16)
        n1169 = Multiply(x="Duty Frequency (ON 1/N cycles)", y=w1734) -> (x*y=w1730:u16)
        "Green AI Count" <- w1730
        "Red AI Count" <- w1730
        "Blue AI Count" <- w1730
        n1170 = Subtract(x=w1730, y="Interlace ON count") -> (x-y=w1733:u16)
        n1171 = Multiply(x=w1745, y="Duty Frequency (ON 1/N cycles)") -> (x*y=w1744:u16)
        n1172 = Subtract(x=w1744, y="APD Gate ON Count") -> (x-y=w1743:u16)
        n1173 = local read "DMA Update Period (s)"() -> (w1746:dbl)
        n1174 = Multiply(x="APD Integration Time (s)", y=40000000.0) -> (x*y=w1750:dbl)
        n1175 = Reciprocal(x="APD Integration Time (s)") -> (1/x=→"APD Acq Rate (Hz)":dbl)
        n1176 = To Unsigned Long Integer(number=w1750) -> (unsigned 32bit integer=w1736:u32)
        "APD Int. Count" <- w1736
        n1177 = local read "Number of APDs"() -> (w1729:u8)
        n1178 = Divide(x=w1746, y="APD Integration Time (s)") -> (x/y=w1748:dbl)
        n1179 = Multiply(x=w1729, y=w1748) -> (x*y=w1747:dbl)
        n1180 = local write "APD Samples/FIFO Acq."(w1748) -> ()
        n1181 = local write "APD Elements/DMA read"(w1747) -> ()
        n1182 = xnode "Read/Write Control"("FPGA VI Reference In"=w1728, "Invert APD Gate"="Invert APD Gate", "APD Gate ON Count"="APD Gate ON Count", "APD Gate OFF Count"=w1743, "APD Acq Rate Count"=w1736, "APD Gate Operating Mode"="APD Gate", "APD AO scale factor"="APD AO Scale Factor", "Green interlace ON count"="Interlace ON count", "Green interlace OFF count"=w1733, "Green interlace ON count 2"="Interlace ON count", "Green interlace OFF count 2"=w1733, "Green FB Count"=w1730, "Red interlace ON count"="Interlace ON count", "Red interlace OFF count"="Interlace OFF count", "Blue ON count (AO)"="Interlace ON count", "Blue OFF count (AO)"="Interlace OFF count", "Blue interlace OFF count (D)"="Interlace OFF count", "Blue interlace ON count (D)"="Interlace ON count") -> ("error out"=w1752:errorcluster)  [unwired: 1 in, 1 out]
      }
      event "Neg. TTrig FPGA": Value Change {
        n1183 = event-data() -> ()  [unwired: 7 out]
        n1184 = xnode "Read/Write Control"("FPGA VI Reference In"=w1753, "TTrig Negate Pos"="Neg. TTrig FPGA") -> ()  [unwired: 1 in, 2 out]
      }
      event "Test ttrig": Value Change {
        n1185 = event-data() -> ()  [unwired: 7 out]
        n1186 = xnode "Read/Write Control"("FPGA VI Reference In"=w1755, "TTrig?"=TRUE) -> ("error out"=w1757:errorcluster)  [unwired: 1 in, 1 out]
      }
      event "Number of F/B Scans (AOD)", "Scan Speed (nm/s)", "Scan BD", "Initial delta (MHz)", "Step Size (nm)", "Scan Range (nm)": Value Change {
        w1821 = 123.0  # AOM cal (nm/MHz)
        n1187 = event-data() -> ()  [unwired: 7 out]
        n1188 = local read "BD 1 Frequency 1 (MHz)"() -> (w1804:dbl)
        n1189 = local read "AOM X Cal (nm/MHz)"() -> (w1796:dbl)
        n1190 = local read "X RF Frequency Limits (MHz)"() -> (w1808:T18)
        n1191 = local read "Y RF Frequency Limits (MHz)"() -> (w1805:T18)
        n1192 = local read "BD 2 Frequency 1 (MHz)"() -> (w1810:dbl)
        n1193 = Negate(x="Scan Range (nm)") -> (-x=w1774:dbl)
        n1194 = Divide(x=w1774, y=w1796) -> (x/y=w1778:dbl)
        n1195 = Select(t=w1808, s="Scan BD", f=w1805) -> (s? t:f=w1807:T18)
        n1196 = Select(t=w1804, s="Scan BD", f=w1810) -> (s? t:f=w1809:dbl)
        n1197 = Unbundle By Name(w1807) -> ("Maximum"=w1816:dbl, "Minimum"=w1815:dbl)
        n1198 = Add(x=w1778, y=w1809) -> (x+y=w1813:dbl)
        n1199 = Divide(x=w1774, y="Step Size (nm)") -> (x/y=w1793:dbl)
        n1200 = Divide(x="Step Size (nm)", y=w1796) -> (x/y=w1802:dbl)
        n1201 = Absolute Value(x=w1793) -> (abs(x)=w1777:dbl)
        n1202 = Sign(1:w1774) -> (0:w1775:dbl)
        n1203 = In Range and Coerce(upper limit=w1816, x=w1813, lower limit=w1815) -> (coerced(x)=w1812:dbl, In Range?=w1814:bool)
        n1204 = To Unsigned Quad Integer(1:w1777) -> (0:w1792:u64)
        "Scan steps (AOD)" <- w1792
        n1205 = call "IR AOM freq to word.vi"("Frequency In (MHz)"=w1802) -> ("Frequency Word Out (double)"=w1799:dbl)
        n1206 = Multiply(x=w1775, y=w1799) -> (x*y=w1776:dbl)
        n1207 = Subtract(x=w1813, y=w1812) -> (x-y=w1811:dbl)
        n1208 = To Quad Integer(1:w1776) -> (0:w1798:i64)
        "Incr. int (AOD)" <- w1798
        n1209 = Subtract(x=w1778, y=w1811) -> (x-y=w1797:dbl)
        "Scan Range (MHz)" <- w1797
        n1210 = Select(t=w1778, s=w1814, f=w1797) -> (s? t:f=w1817:dbl)
        n1211 = Multiply(x=w1797, y=w1796) -> (x*y=w1795:dbl)
        n1212 = Decrement(x=w1792) -> (x-1=w1845:u64)
        n1213 = Negate(x=w1795) -> (-x=w1791:dbl)
        n1214 = local write "Scan Range (nm)"(w1791) -> ()
        n1215 = Divide(x=w1817, y=w1845) -> (x/y=w1801:dbl)
        "Scan Increment (MHz)" <- w1801
        n1216 = call "IR AOM freq to word.vi"("Frequency In (MHz)"=w1801) -> ("Frequency Word Out (double)"=w1800:dbl)
        n1217 = Divide(x="Step Size (nm)", y="Scan Speed (nm/s)") -> (x/y=w1788:dbl)
        n1218 = To Quad Integer(1:w1800) -> ()  [unwired: 1 out]
        n1219 = local read "Number Interlace Sets"() -> (w1772:u8)
        n1220 = local read "AI Count (ticks)"() -> (w1773:u16)
        n1221 = local read "Total Counts (ticks)"() -> (w1771:u16)
        n1222 = local read "# Samples/trap"() -> (w1803:u32)
        n1223 = Multiply(x=w1773, y=w1772) -> (x*y=w1770:u16)
        n1224 = Divide(x=w1771, y=w1770) -> (x/y=w1769:dbl)
        n1225 = Select(t=w1804, s="Scan BD", f=w1810) -> (s? t:f=w1842:dbl)
        "Initial freq. (MHz)" <- w1842
        n1226 = Add(x=w1817, y=w1842) -> (x+y=→"Final freq. (MHz)":dbl)
        n1227 = Divide(x=w1771, y=40000000.0) -> (x/y=w1787:dbl)
        n1228 = Divide(x=w1788, y=w1787) -> (x/y=w1786:dbl)
        n1229 = To Unsigned Quad Integer(1:w1786) -> (0:w1761:u64)
        n1230 = Quotient & Remainder(x=w1761, y=u64 2) -> (x-y*floor(x/y)=w1765:u64)  [unwired: 1 out]
        n1231 = Equal?(x=w1765, y=u64 0) -> (x = y?=w1763:bool)
        n1232 = Decrement(x=w1761) -> (x-1=w1762:u64)
        n1233 = Select(t=w1761, s=w1763, f=w1762) -> (s? t:f=w1760:u64)
        "Cycles/step (AOD)" <- w1760
        n1234 = xnode "Read/Write Control"("FPGA VI Reference In"=w1759, "Scan steps"=w1792, "Number of scans"="Number of F/B Scans (AOD)", "Cycles per step"=w1760, "Scan freq.  increment"=w1798, "Scan BD"="Scan BD") -> ("error out"=w1851:errorcluster)  [unwired: 1 in, 1 out]
        n1235 = Multiply(x=w1792, y=w1760) -> (x*y=w1846:u64)
        n1236 = Multiply(x=w1846, y=u64 2) -> (x*y=w1768:u64)
        n1237 = Multiply(x=w1769, y=w1768) -> (x*y=w1767:dbl)
        "Data points/scan (f/b)" <- w1767
        n1238 = Multiply(x=w1767, y="Number of F/B Scans (AOD)") -> (x*y=w1849:dbl)
        "Data points/scans" <- w1849
        n1239 = Divide(x=w1849, y=w1803) -> (x/y=→"N sets should be saved":dbl)
        n1240 = Multiply(x=w1846, y=w1787) -> (x*y=w1785:dbl)
        "Time/Scan (s) (AOD)" <- w1785
        n1241 = Select(t=w1817, s="Scan BD", f=0.0) -> (s? t:f=w1843:dbl)
        n1242 = Select(t=0.0, s="Scan BD", f=w1817) -> (s? t:f=w1839:dbl)
        n1243 = local read "BD 2 Frequency 2 (MHz)"() -> (w1835:dbl)
        n1244 = local read "BD 1 Frequency 2 (MHz)"() -> (w1838:dbl)
        n1245 = Add(x=w1839, y=w1810) -> (x+y=w1836:dbl)
        n1246 = Add(x=w1804, y=w1843) -> (x+y=w1837:dbl)
        n1247 = Multiply(x=w1785, y=2.0) -> (x*y=w1784:dbl)
        n1248 = Multiply(x=w1784, y="Number of F/B Scans (AOD)") -> (x*y=w1781:dbl)
        n1249 = Divide(x=w1781, y=60.0) -> (x/y=→"Time to Finish All (min)":dbl)
        n1250 = Add(x="Trap 2 Bead Size (nm)", y="Trap 1 Bead Size (nm)") -> (x+y=w1825:dbl)
        n1251 = Divide(x=w1825, y=2.0) -> (x/y=w1819:dbl)
        n1252 = local read "Initial delta (MHz)"() -> (w1822:dbl)
        n1253 = Subtract(x=w1836, y=w1835) -> (x-y=w1833:dbl)
        n1254 = Subtract(x=w1837, y=w1838) -> (x-y=w1834:dbl)
        n1255 = Square(x=w1833) -> (x^2=w1832:dbl)
        n1256 = Square(x=w1834) -> (x^2=w1831:dbl)
        n1257 = Add(x=w1831, y=w1832) -> (x+y=w1830:dbl)
        n1258 = Square Root(x=w1830) -> (sqrt(x)=w1829:dbl)
        "Final delta (MHz)" <- w1829
        n1259 = Multiply(x=w1821, y=w1829) -> (x*y=w1828:dbl)
        n1260 = Multiply(x=w1822, y=w1821) -> (x*y=w1820:dbl)
        n1261 = Subtract(x=w1820, y=w1819) -> (x-y=→"Initial sep (nm)":dbl)
        n1262 = Subtract(x=w1828, y=w1819) -> (x-y=→"Final sep (nm)":dbl)
      }
      event "Freq or Amp switch first", "Swap F1 and F2", "Freq switch delay", "Amp switch delay": Value Change {
        n1263 = event-data() -> ()  [unwired: 7 out]
        n1264 = local read "Amp switch delay"() -> (w1853:u16)
        n1265 = local read "Swap F1 and F2"() -> (w1854:bool)
        n1266 = xnode "Read/Write Control"("FPGA VI Reference In"=w1852, "Swap F1 and F2"=w1854, "Amp switch delay"=w1853) -> ("error out"=w1855:errorcluster)  [unwired: 1 in, 1 out]
      }
      event "Scan steps (MCL)", "Number of scans (MCL)", "Scan Range (V)\n(of steps)", "2D or 1D Scan", "N APD Samp/step", "Fast Scan Dir", "Continuous MCL Scanning", "Scan lines (y)": Value Change {
        w1858 = 32767.0 ("y")
        n1267 = event-data() -> ()  [unwired: 7 out]
        n1268 = Select(t="Scan lines (y)", s="2D or 1D Scan", f="Number of scans (MCL)") -> (s? t:f=w1863:u64)
        n1269 = Decrement(x="Scan steps (MCL)") -> (x-1=w1879:u64)
        n1270 = Divide(x="Scan Range (V)\n(of steps)", y=w1879) -> (x/y=w1878:dbl)
        "Desired Scan Incr (V)" <- w1878
        n1271 = local read "APD Integration Time (s)"() -> (w1871:dbl)
        n1272 = Multiply(x=w1878, y=w1858) -> (x*y=w1887:dbl)
        n1273 = Divide(x=w1887, y=10.0) -> (x/y=w1877:dbl)
        "Desired incr (int)" <- w1877
        n1274 = local read "Update Count (MCL)"() -> (w1883:u32)
        n1275 = Round Toward -Infinity(1:w1877) -> (0:w1886:dbl)
        n1276 = To Word Integer(number=w1886) -> (16bit integer=w1861:i16)
        "Actual Incr. int (MCL)" <- w1861
        n1277 = Multiply(x=w1871, y=40000000.0) -> (x*y=w1884:dbl)
        n1278 = Divide(x=w1884, y=w1883) -> (x/y=w1882:dbl)
        n1279 = Multiply(x=i16 10, y=w1861) -> (x*y=w1859:i16)
        n1280 = Multiply(x="N APD Samp/step", y=w1882) -> (x*y=w1881:dbl)
        "Cycles/step (MCL)" <- w1881
        n1281 = Divide(x=w1859, y=w1858) -> (x/y=→"Actual MCL Inc (V)":dbl)
        n1282 = Multiply(x="N APD Samp/step", y="Scan steps (MCL)") -> (x*y=w1873:dbl)
        n1283 = local read "APD Samples/FIFO Acq."() -> (w1870:dbl)
        n1284 = Multiply(x=w1873, y=u64 2) -> (x*y=w1872:dbl)
        "Data points/scan (f+b)" <- w1872
        n1285 = Multiply(x=w1872, y=w1863) -> (x*y=w1890:dbl)
        "Data points/scans (MCL)" <- w1890
        n1286 = Multiply(x=w1871, y=w1872) -> (x*y=w1864:dbl)
        "Time/f+b scan (s) (MCL)" <- w1864
        n1287 = Divide(x=w1890, y=w1870) -> (x/y=→"N sets should be saved (MCL)":dbl)
        n1288 = Multiply(x=w1864, y=w1863) -> (x*y=→"Total Time (s)":dbl)
        n1289 = Not(x="Fast Scan Dir") -> (.not. x?=w1868:bool)
        n1290 = xnode "Read/Write Control"("FPGA VI Reference In"=w1856, "Scan steps (MCL)"="Scan steps (MCL)", "Number of scans (MCL)"=w1863, "Cycles per step (MCL)"=w1881, "Scan freq.  increment (MCL)"=w1861, "1D or 2D Scan?"="2D or 1D Scan", "MCL Scan Axis"=w1868, "Cont. Scan (MCL)"="Continuous MCL Scanning") -> ("error out"=w1892:errorcluster)  [unwired: 1 in, 1 out]
      }
      event "Read Cal": Value Change {
        w1904 = 1000.0 ("y")
        n1291 = event-data() -> ()  [unwired: 7 out]
        n1292 = local read "Save file name"() -> (w1923:path)
        n1293 = local write "Read Cal"(FALSE ("Read Cal")) -> ()
        n1294 = Strip Path(path=w1923) -> (stripped path=w1922:path)  [unwired: 1 out]